vi "Main.vi"() -> ()   [LabVIEW 2020]
uses:
  System.Windows.Forms
  Global_Variable/Global.vi
  Global_Variable/A131258.vi
  Database/Global1.vi
  <userlib>/_MGI/Menu Building/MenuTypes/MenuStrip/MGI_MenuStrip.lvclass
  <userlib>/_MGI/Menu Building/MenuItemStatusChange/MGI_MenuItemStatusChange.lvclass
  Libraries/S7/S7.lvlib
panel:
  out "右加载扭矩":dbl format="%#.3f Nm"
  out "左空载扭矩":dbl format="%#.3f Nm"
  out "上序状态":string
  in  "表格控件":string[][](table)
  in  "Andon":enum32{"未选择", "缺料报警", "质量报警", "故障报警"}(radio)
  out "PLC":bool
  in  "菜单":refnum<k24>(container)
  out "试验计时":u16
  out "工位传感器码":string
  out "生产数量":i32
  out "合格数量":i32
  out "userStatus":string caption="用户状态"
  out "userName":string caption="用户名"
  out "connectionMode":string caption="联机类型"
  out "产品型号":string
  in  "更换产品":refnum<vi>
  out "提示信息":string
  out "错误":bool
  out "时间字符串":string
  out "日期字符串":string
  out "自动":bool
  # "芯轴分总成磨合台"
  # "试验项目"
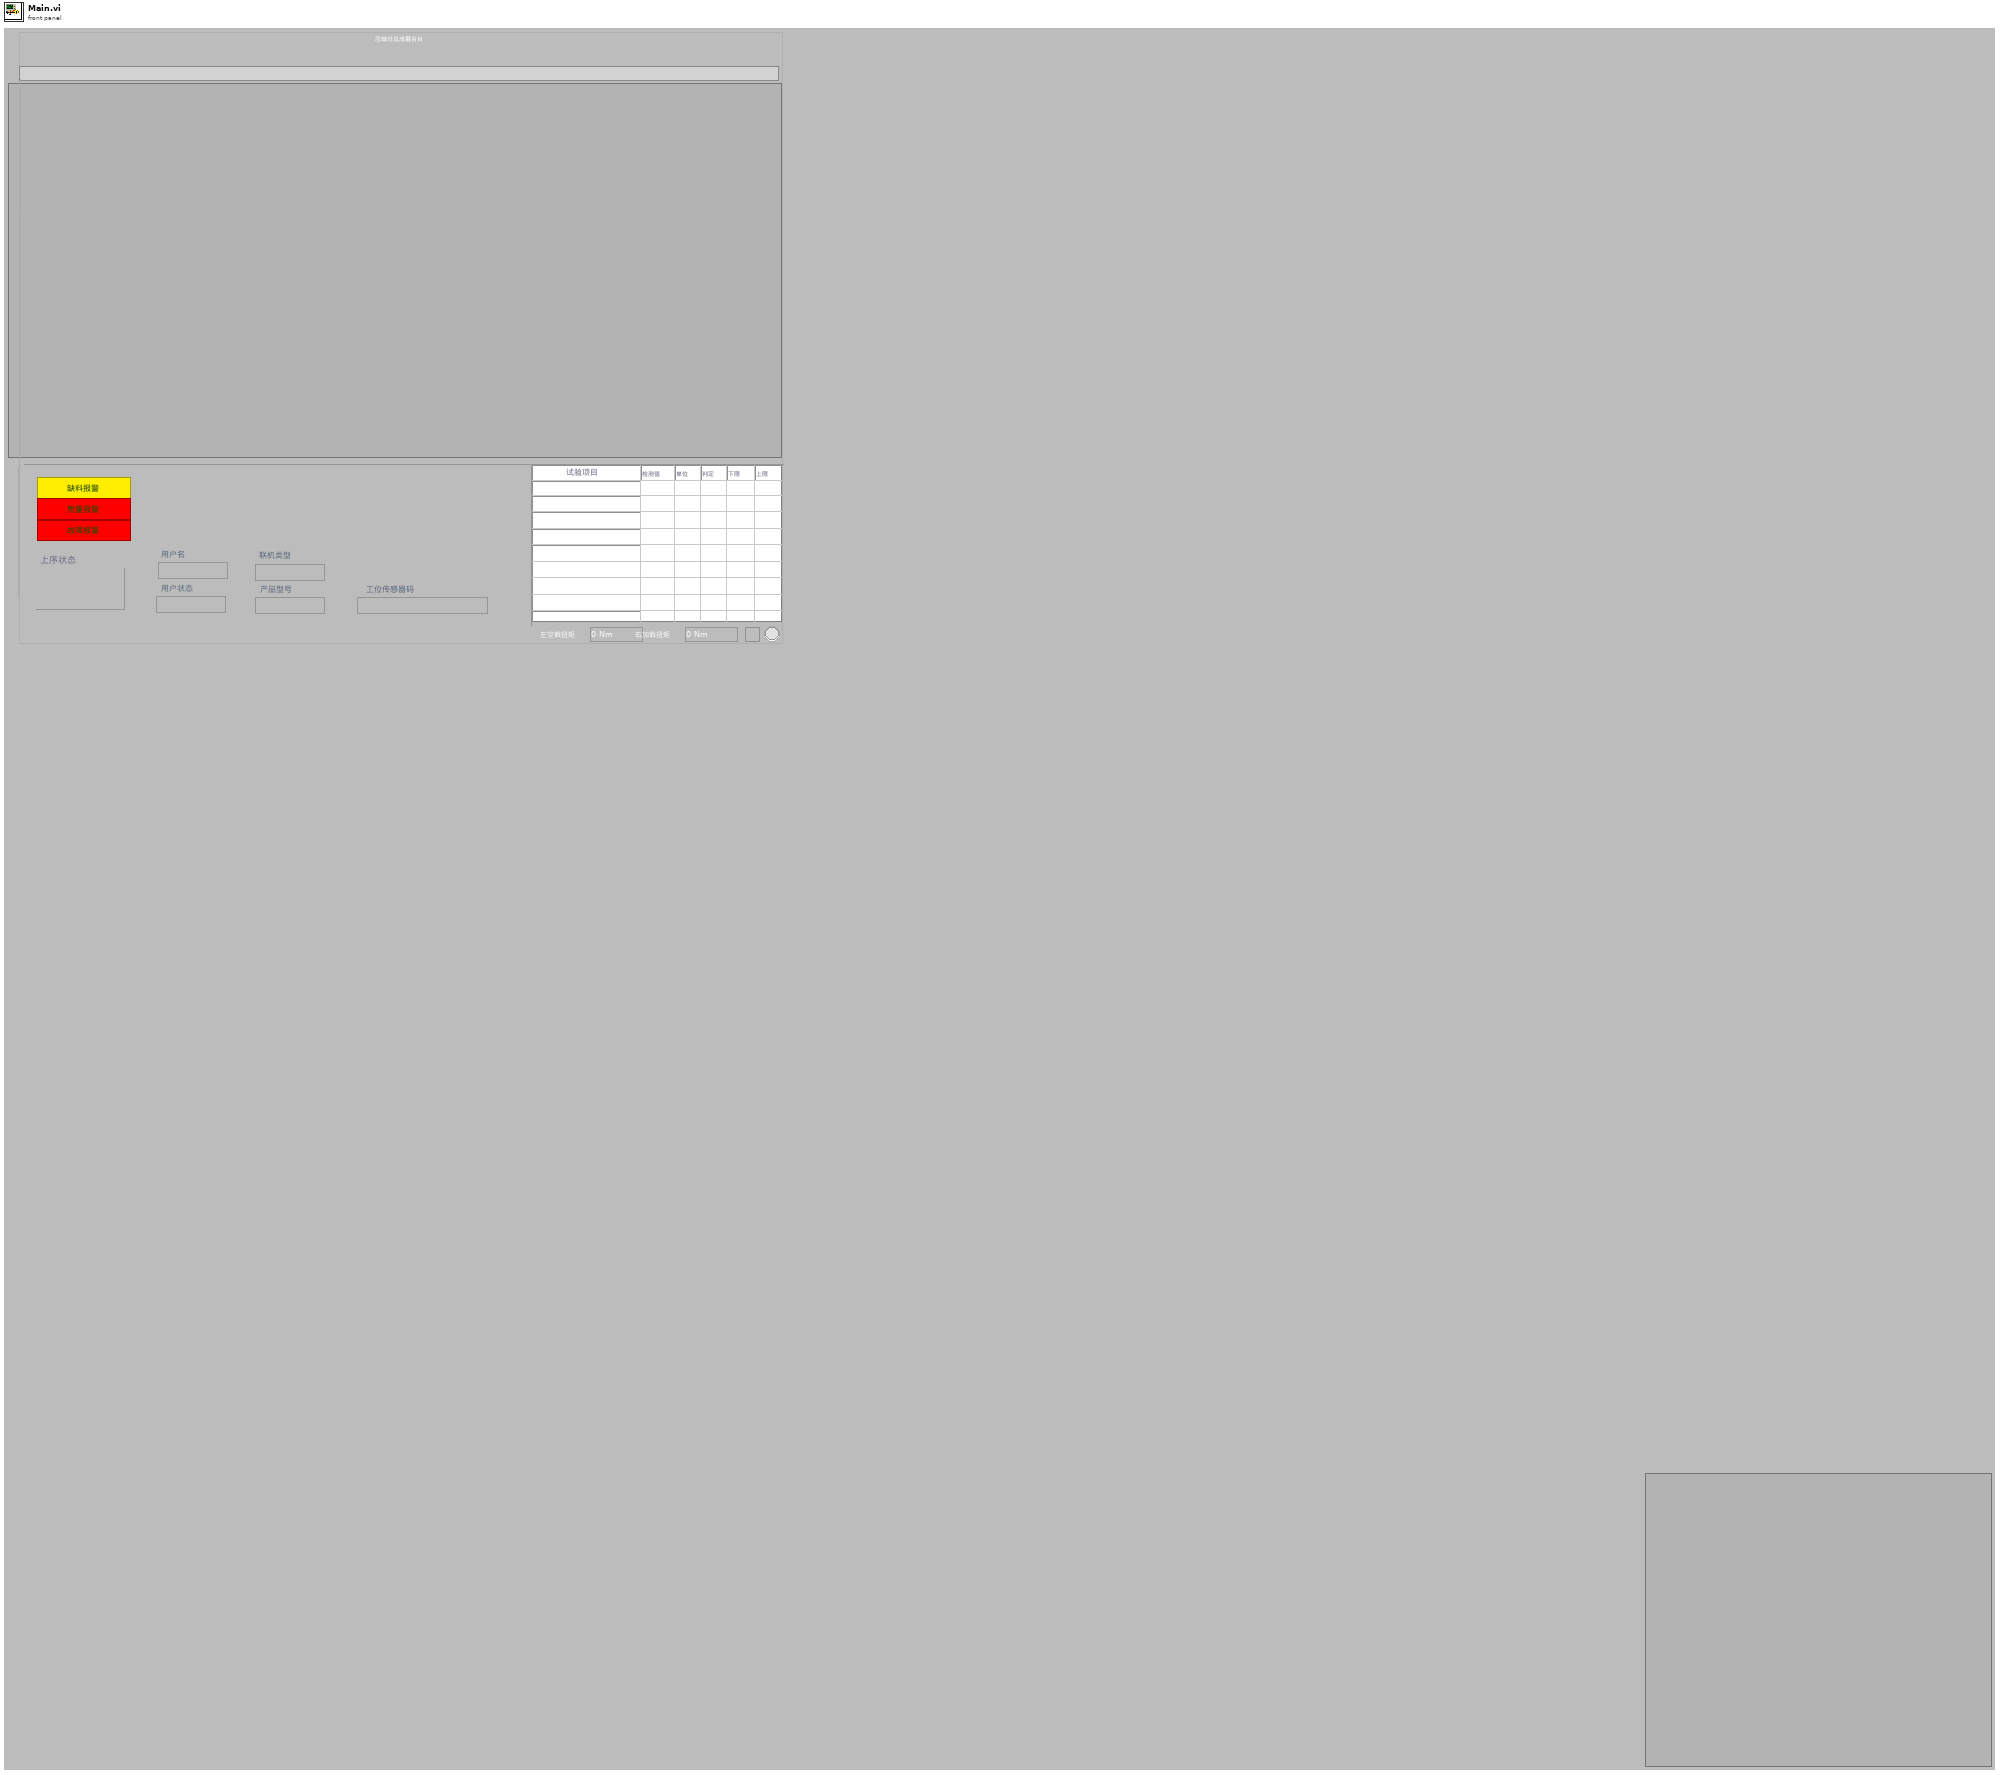
[diagram p1: front panel]
types:
  T1 = typedef "S7.lvlib/Broadcast Events--cluster.ctl" = cluster{"Module Did Init":refnum<user-event>, "Status Updated":refnum<user-event>, "Error Reported":refnum<user-event>, "Module Did Stop":refnum<user-event>, "Update Module Execution Status":refnum<user-event>}
  T2 = enum32{"Invalid", "Standard", "Closed", "Hidden", "Minimized", "Maximized"}
  T3 = cluster{"设备名称":string, "操作人员":string, "设备状态":enum16{"设备离线", "设备正常", "设备缺料", "设备故障", "质量报警"}, "附加信息":string}
  T4 = enum32{"invalid app kind", "Development System", "Run Time System", "Student Edition", "Embedded LabVIEW", "Evaluation", "Custom"}
  T5 = cluster{"左平均扭矩":cluster{"正转":dbl, "反转":dbl}, "左矩波动":cluster{"正转":dbl, "反转":dbl}, "左空载":cluster{"正转":dbl, "反转":dbl}, "右平均扭矩":cluster{"正转":dbl, "反转":dbl}, "右扭矩波动":cluster{"正转":dbl, "反转":dbl}, "右空载":cluster{"正转":dbl, "反转":dbl}, "扭矩对称":cluster{"左":dbl, "右":dbl}, "左零点漂移":cluster{"正":dbl, "反":dbl}, "右零点漂移":cluster{"正":dbl, "反":dbl}}
  T6 = cluster{"用户编号":string, "用户名":string, "用户密码(密文)":string, "用户权限":string}
  T7 = cluster{"Core":cluster{"Current VI Reference":refnum<vi>, "Close Panel on Exit?":bool}, "Your Boolean data":bool, "Your string data":string}
  T8 = cluster{"Current VI Reference":refnum<vi>, "Close Panel on Exit?":bool}
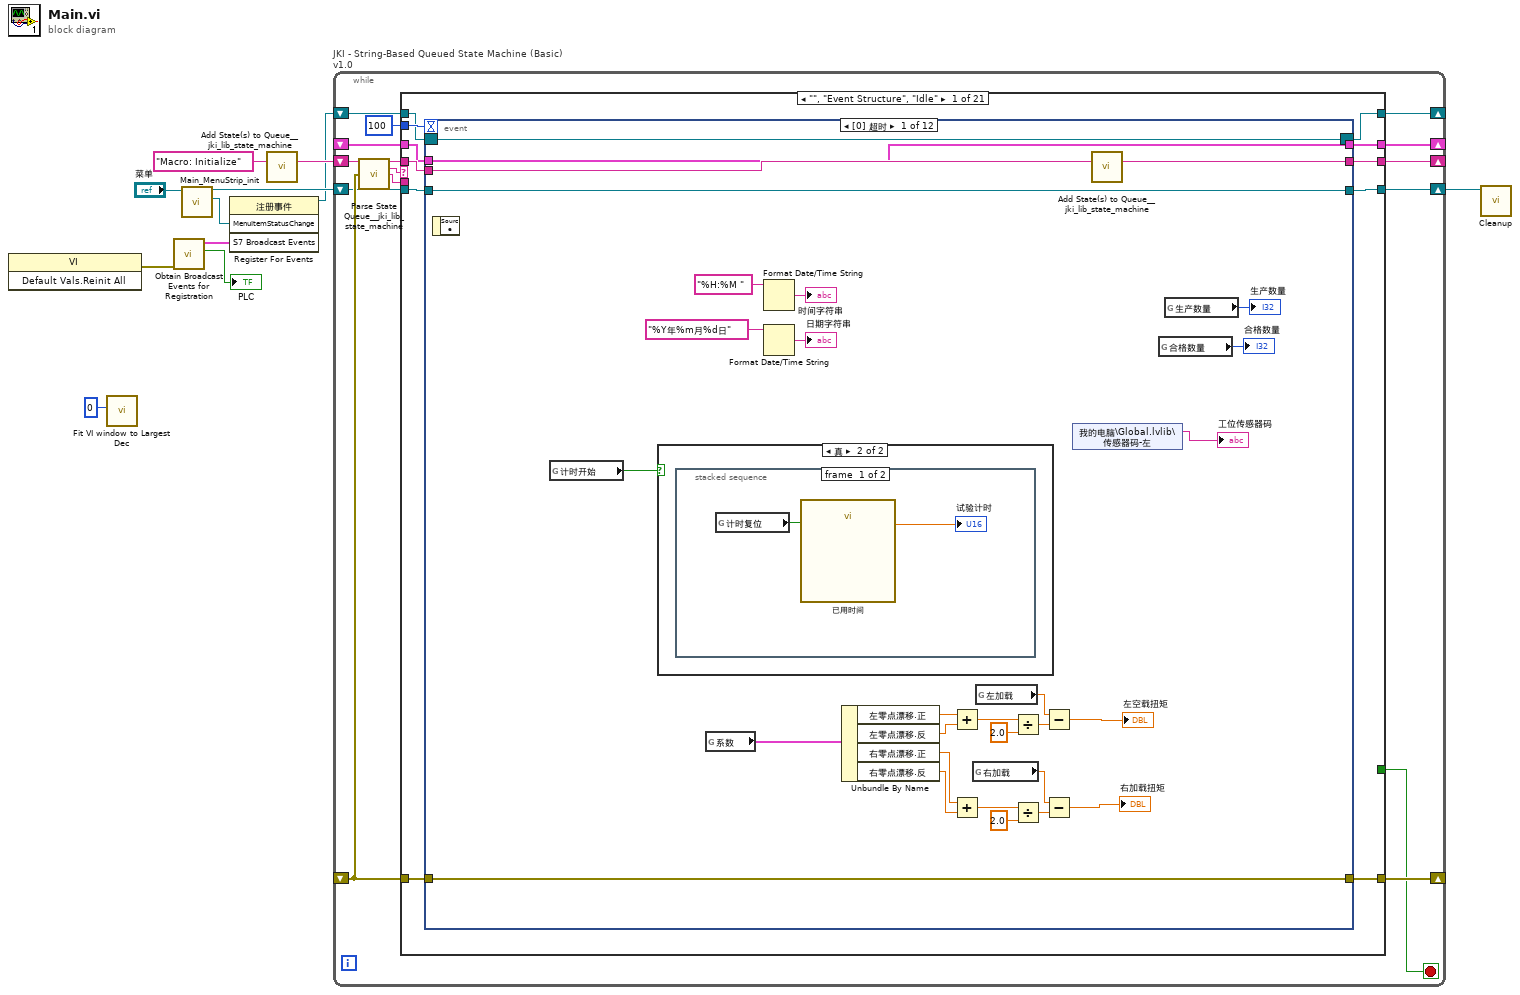
[diagram p0: block diagram]
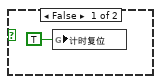
[diagram p2: hidden frame]
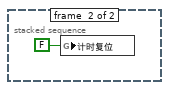
[diagram p3: hidden frame]
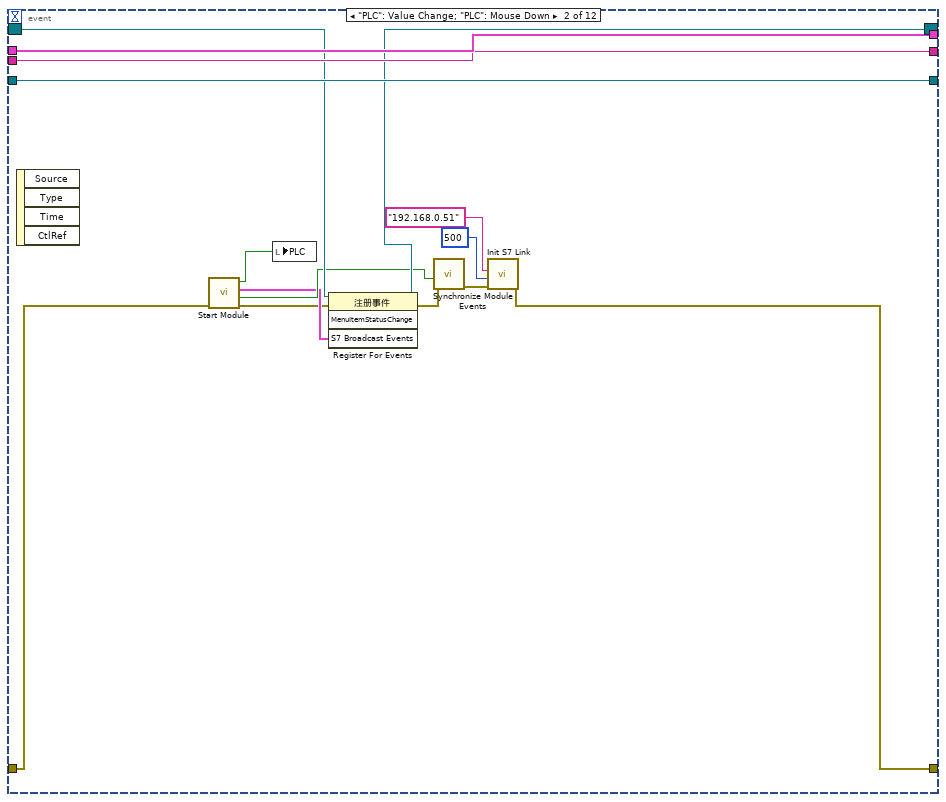
[diagram p4: hidden frame]
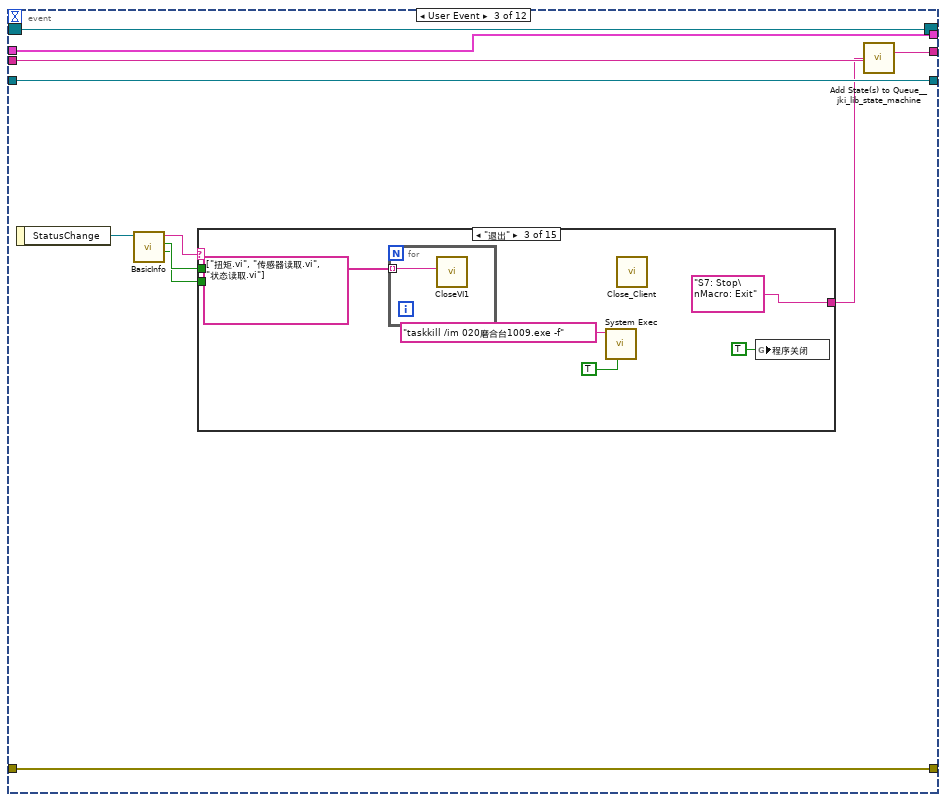
[diagram p5: hidden frame]
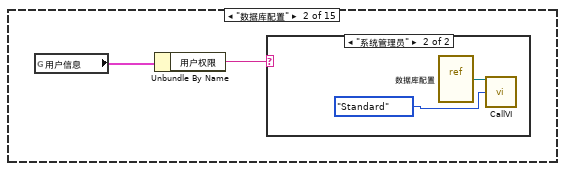
[diagram p7: hidden frame]
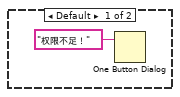
[diagram p8: hidden frame]
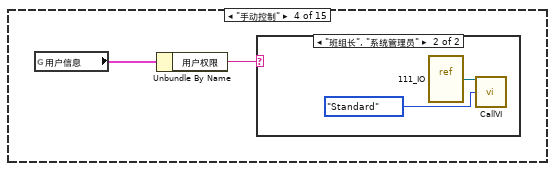
[diagram p9: hidden frame]
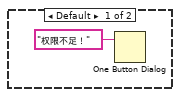
[diagram p10: hidden frame]
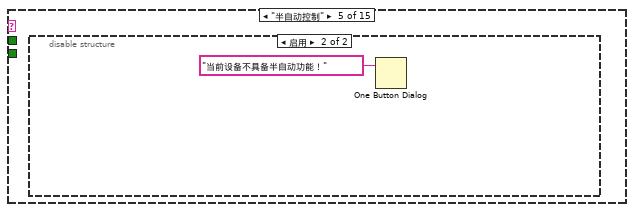
[diagram p11: hidden frame]
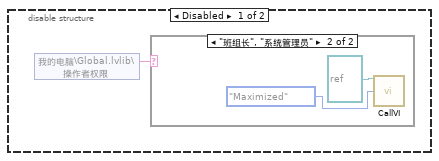
[diagram p12: hidden frame]
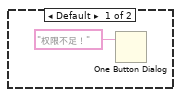
[diagram p13: hidden frame]
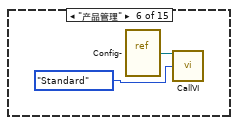
[diagram p14: hidden frame]
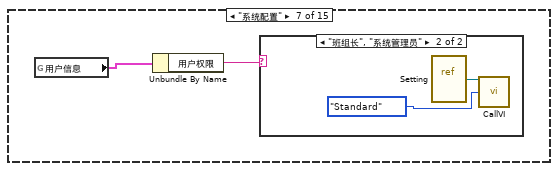
[diagram p15: hidden frame]
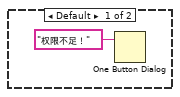
[diagram p16: hidden frame]
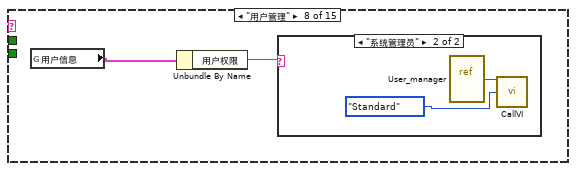
[diagram p17: hidden frame]
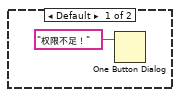
[diagram p18: hidden frame]
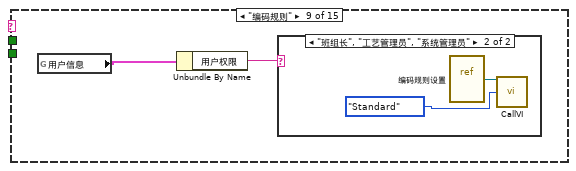
[diagram p19: hidden frame]
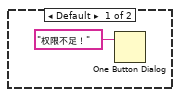
[diagram p20: hidden frame]
diagram:
  n1 = invoke class="VI" method="Default Vals.Reinit All"() -> (error out=w4:errorcluster)  [unwired: 3 in, 2 out]
  n2 = call "Fit VI window to Largest Dec.vi"("border spacing (2 px)"=0) -> ()  [unwired: 5 in, 2 out]
  n3 = call "Obtain Broadcast Events for Registration.vi"("error in (no error)"=w4) -> ("Already running?"=→"PLC":bool, "S7 Broadcast Events"=w6:T1)  [unwired: 8 in, 1 out]
  n4 = call "Main_MenuStrip_init.vi"("MenuStrip"="菜单") -> ("MenuItemStatusChange"=w3:refnum<user-event>, "Menu out"=w8:refnum<class "MGI_MenuStrip.lvclass">)  [unwired: 9 in]
  n5 = register-events(w3, w6) -> (reference out=w2:refnum<event-registration>)  [unwired: 2 in, 1 out]
  n6 = call <vilib>:"Add State(s) to Queue__jki_lib_state_machine.vi"("State(s) in (\"\")"="Macro: Initialize") -> ("States Out"=w11:string)  [unwired: 14 in]
  n7 = while "JKI - String-Based Queued State Machine (Basic) v1.0" {
    shift-right: [w20] -> _
    shift-left: _ -> [w19]
    shift-right: [w22] -> _
    shift-left: _ -> [w17]
    shift-right: [w21] -> _
    shift-left: w11 -> [w23]
    shift-right: [w15] -> w7
    shift-left: w8 -> [w16]
    shift-right: [w13] -> _
    shift-left: w2 -> [w12]
    stop <- w14 stop-if-true
    n8 = call <vilib>:"Parse State Queue__jki_lib_state_machine.vi"("State Queue"=w23, "Error In (no error)"=w17) -> ("Remaining States"=w25:string, "Current State"=w26:string, "Arguments"=w24:string)  [unwired: 11 in]
    n9 = case shown="\"\", \"Event Structure\", \"Idle\"" w26 {
      selector: w26 -> [_ _ w249 _ _ _ _ _ _ _ _ _ _ _ _ _ _ _ _ _ _]
      tunnel: w25 -> [w37 w246 w253 w273 w281 w289 w295 w299 w305 w314 w325 w333 w339 w349 w373 w409 w417 w430 w458 w465 w478]
      tunnel: w24 -> [_ _ _ _ _ _ _ _ _ _ _ _ _ _ _ _ w412 w424 _ _ _]
      tunnel: w19 -> [w35 w243 w251 w264 w278 w287 w292 w300 w308 w311 _ w328 w336 w347 w371 w406 w415 w426 w455 w462 w475]
      tunnel: [w34 w244 w255 w270 errorcluster {"status"=FALSE, "code"=0, "source"=""} ("error out") w286 w293 w297 w303 w312 w322 w329 w337 w346 w369 w407 w413 w427 w456 w463 w476] -> w22
      tunnel: w17 -> [w33 w244 w254 w270 w277 w286 w293 w297 w304 w312 w322 w330 w337 w340 w369 w407 w414 w428 w456 w463 w476]
      tunnel: [w36 w245 w252 w272 w280 w288 w294 w299 w306 w313 w324 w332 w338 w348 w372 w408 w416 w429 w457 w464 w477] -> w21
      tunnel: [w32 w243 w251 w271 w278 w287 w292 w300 w308 w311 w323 w328 w336 w347 w371 w406 w415 w426 w455 w462 w475] -> w20
      tunnel: 100 ("Timeout") -> [w31 _ _ _ _ _ _ _ _ _ _ _ _ _ _ _ _ _ _ _ _]
      tunnel: w16 -> [w30 w242 w248 w261 w275 w285 w291 w298 w307 w310 w317 w327 w335 w345 w370 w405 w411 w423 w454 w460 w468]
      tunnel: [w29 w242 w248 w261 w275 w285 w291 w298 w307 w310 w317 w327 w335 w345 w370 w405 w411 w423 w454 w460 w468] -> w15
      tunnel: [_ _ _ _ _ TRUE _ _ _ _ _ _ _ _ _ _ _ _ _ _ _] -> w14
      tunnel: [w27 w241 w247 w260 w274 w283 w290 w301 w302 w309 w318 w326 w334 w344 w368 w402 w410 w422 w453 w459 w467] -> w13
      tunnel: w12 -> [w28 w241 w247 w260 w274 w283 w290 w301 w302 w309 w318 w326 w334 w344 w368 w402 w410 w422 w453 w459 w467]
      frame "", "Event Structure", "Idle" {
        n10 = event shown="[0] 超时" {
          selector: w28 -> [w56 w80 w86 w156 w163 w170 w177 w191 w200 w208 w217 _]
          dyn-events: [w56 w79 w86 w156 w163 w170 w177 w191 w200 w208 w217 _] -> w27
          timeout: w31 -> [_ _ _ _ _ _ _ _ _ _ _ _]
          tunnel: w37 -> [w66 w84 w95 w157 w164 w173 w180 w188 w204 w215 w219 w235]
          tunnel: [w65 w84 w93 w158 w165 w174 w181 w189 w205 w214 w220 w235] -> w36
          tunnel: w35 -> [w64 w85 w94 w160 w168 w175 w182 w190 w206 w212 w222 w236]
          tunnel: [w57 w81 w96 w161 w166 w171 w183 w186 w203 w213 w221 w233] -> w34
          tunnel: w33 -> [w57 w82 w96 w161 w166 w171 w184 w186 w203 w213 w221 w233]
          tunnel: [w64 w85 w94 w160 w168 w175 w182 w190 w206 w212 w222 w236] -> w32
          tunnel: w30 -> [w55 w83 w89 w159 w167 w172 w179 w187 _ _ _ w234]
          tunnel: [w55 w83 w89 w159 w167 w172 w179 w187 _ _ _ w234] -> w29
          event Timeout {
            n11 = event-data() -> ()  [unwired: 1 in, 1 out]
            n12 = global read "Global.vi" "计时开始"() -> (w54:bool)
            n13 = case shown="真" w54 {
              frame False {
                n14 = global write "Global.vi" "计时复位"(TRUE ("计时复位")) -> ()
              }
              frame True {
                n15 = stacked-sequence {
                  frame #0 {
                    n16 = global read "Global.vi" "计时复位"() -> (w68:bool)
                    n17 = call "已用时间"("Reset"=w68) -> ("Elapsed Time (s)"=→"试验计时":dbl)  [unwired: 11 in, 7 out]
                  }
                  frame #1 {
                    n18 = global write "Global.vi" "计时复位"(FALSE ("计时复位")) -> ()
                  }
                }
              }
            }
            n19 = global read "A131258.vi" "系数"() -> (w38:T5)
            n20 = Format Date/Time String(time format string (%c)="%H:%M ") -> (date/time string=→"时间字符串":string)  [unwired: 2 in]
            n21 = Format Date/Time String(time format string (%c)="%Y年%m月%d日") -> (date/time string=→"日期字符串":string)  [unwired: 2 in]
            n22 = Unbundle By Name(w38) -> ("左零点漂移.正"=w39:dbl, "左零点漂移.反"=w40:dbl, "右零点漂移.正"=w47:dbl, "右零点漂移.反"=w48:dbl)
            n23 = Add(x=w39, y=w40) -> (x+y=w41:dbl)
            n24 = Add(x=w47, y=w48) -> (x+y=w46:dbl)
            n25 = global read "全局2.vi" "右加载"() -> (w49:dbl)
            n26 = global read "全局1.vi" "左加载"() -> (w43:dbl)
            n27 = Divide(x=w41, y=2.0) -> (x/y=w42:dbl)
            n28 = Divide(x=w46, y=2.0) -> (x/y=w45:dbl)
            n29 = Subtract(x=w43, y=w42) -> (x-y=→"左空载扭矩":dbl)
            n30 = Subtract(x=w49, y=w45) -> (x-y=→"右加载扭矩":dbl)
            n31 = shared-variable "我的电脑\\Global.lvlib\\传感器码-左"() -> (→"工位传感器码":string)  [unwired: 1 in, 1 out]
            n32 = call <vilib>:"Add State(s) to Queue__jki_lib_state_machine.vi"("State(s) in (\"\")"=w66) -> ("States Out"=w65:string)  [unwired: 14 in]
            n33 = global read "Global.vi" "合格数量"() -> (→"合格数量":i32)
            n34 = global read "Global.vi" "生产数量"() -> (→"生产数量":i32)
          }
          event "PLC": Value Change; "PLC": Mouse Down {
            n35 = event-data() -> ()  [unwired: 1 in, 4 out]
            n36 = call "Start Module.vi"("error in (no error)"=w82) -> ("error out"=w75:errorcluster, "Wait for Event Sync?"=w78:bool, "S7 Broadcast Events"=w77:T1, "Module Was Already Running?"=w76:bool)  [unwired: 7 in]
            n37 = local write "PLC"(w76) -> ()
            n38 = register-events(reference=w80, error in=w75, w77) -> (reference out=w79:refnum<event-registration>, error out=w74:errorcluster)  [unwired: 1 in]
            n39 = call "Synchronize Module Events.vi"("error in (no error)"=w74, "Wait for Event Sync?"=w78) -> ("error out"=w71:errorcluster)  [unwired: 9 in]
            n40 = call "Init S7 Link.vi"("error in (no error)"=w71, "超时"=500, "IP"="192.168.0.51") -> ("error out"=w81:errorcluster)  [unwired: 8 in]
          }
          event User Event {
            n41 = event-data() -> ("StatusChange"=w87:refnum<class "MGI_MenuItemStatusChange.lvclass">)  [unwired: 1 in]
            n42 = call <userlib>:"BasicInfo.vi"("MGI_MenuItemStatusChange in"=w87) -> ("Enabled?"=w90:bool, "Checked?"=w91:bool, "Tag"=w92:string)  [unwired: 7 in, 1 out]
            n43 = case shown="\"退出\"" w92 {
              tunnel: w91 -> [_ _ _ _ _ _ _ _ _ _ _ _ _ _ _]
              tunnel: w90 -> [_ _ _ _ _ _ _ _ _ _ _ _ _ _ _]
              tunnel: [_ _ "S7: Stop\nMacro: Exit" _ _ _ _ _ _ _ _ _ _ _ _] -> w88
              frame "假", Default {
              }
              frame "数据库配置" {
                n44 = global read "Global1.vi" "用户信息"() -> (w97:T6)
                n45 = Unbundle By Name(w97) -> ("用户权限"=w98:string)
                n46 = case shown="\"系统管理员\"" w98 {
                  frame Default {
                    n47 = One Button Dialog(message="权限不足！" ("消息")) -> ()  [unwired: 1 in, 1 out]
                  }
                  frame "系统管理员" {
                    n48 = vi-ref "数据库配置.vi"() -> (w101:refnum<vi>)
                    n49 = call "CallVI.vi"("VI引用"=w101, "状态"=T2."Standard") -> ()  [unwired: 11 in, 3 out]
                  }
                }
              }
              frame "退出" {
                n50 = for {
                  tunnel: string[] ["扭矩.vi", "传感器读取.vi", "状态读取.vi"] -> [w107] mode=indexing
                  n51 = call "CloseVI1.vi"("名称或相对路径"=w107) -> ()  [unwired: 10 in, 1 out]
                }
                n52 = call <vilib>:"System Exec.vi"("run minimized? (F)"=TRUE, "command line"="taskkill /im 020磨合台1009.exe -f") -> ()  [unwired: 6 in, 4 out]
                n53 = call "Close_Client.vi"() -> ()  [unwired: 12 in]
                n54 = global write "Global.vi" "程序关闭"(TRUE ("程序关闭")) -> ()
              }
              frame "手动控制" {
                n55 = global read "Global1.vi" "用户信息"() -> (w108:T6)
                n56 = Unbundle By Name(w108) -> ("用户权限"=w109:string)
                n57 = case shown="\"班组长\", \"系统管理员\"" w109 {
                  frame Default {
                    n58 = One Button Dialog(message="权限不足！" ("消息")) -> ()  [unwired: 1 in, 1 out]
                  }
                  frame "班组长", "系统管理员" {
                    n59 = vi-ref "111_IO.vi"() -> (w112:refnum<vi>)
                    n60 = call "CallVI.vi"("VI引用"=w112, "状态"=T2."Standard") -> ()  [unwired: 11 in, 3 out]
                  }
                }
              }
              frame "半自动控制" {
                n61 = disable-structure shown="启用" {
                  frame Disabled {
                    n62 = shared-variable "我的电脑\\Global.lvlib\\操作者权限"() -> (w113:string)  [unwired: 1 in, 1 out]
                    n63 = case shown="\"班组长\", \"系统管理员\"" w113 {
                      frame Default {
                        n64 = One Button Dialog(message="权限不足！" ("消息")) -> ()  [unwired: 1 in, 1 out]
                      }
                      frame "班组长", "系统管理员" {
                        n65 = call "CallVI.vi"("VI引用"=refnum<vi> refnum, "状态"=T2."Maximized") -> ()  [unwired: 11 in, 3 out]
                      }
                    }
                  }
                  frame Enabled {
                    n66 = One Button Dialog(message="当前设备不具备半自动功能！" ("消息")) -> ()  [unwired: 1 in, 1 out]
                  }
                }
              }
              frame "产品管理" {
                n67 = vi-ref "Config-.vi"() -> (w119:refnum<vi>)
                n68 = call "CallVI.vi"("VI引用"=w119, "状态"=T2."Standard") -> ()  [unwired: 11 in, 3 out]
              }
              frame "系统配置" {
                n69 = global read "Global1.vi" "用户信息"() -> (w120:T6)
                n70 = Unbundle By Name(w120) -> ("用户权限"=w121:string)
                n71 = case shown="\"班组长\", \"系统管理员\"" w121 {
                  frame Default {
                    n72 = One Button Dialog(message="权限不足！" ("消息")) -> ()  [unwired: 1 in, 1 out]
                  }
                  frame "班组长", "系统管理员" {
                    n73 = vi-ref "Setting.vi"() -> (w124:refnum<vi>)
                    n74 = call "CallVI.vi"("VI引用"=w124, "状态"=T2."Standard") -> ()  [unwired: 11 in, 3 out]
                  }
                }
              }
              frame "用户管理" {
                n75 = global read "Global1.vi" "用户信息"() -> (w125:T6)
                n76 = Unbundle By Name(w125) -> ("用户权限"=w126:string)
                n77 = case shown="\"系统管理员\"" w126 {
                  frame Default {
                    n78 = One Button Dialog(message="权限不足！" ("消息")) -> ()  [unwired: 1 in, 1 out]
                  }
                  frame "系统管理员" {
                    n79 = vi-ref "User_manager.vi"() -> (w129:refnum<vi>)
                    n80 = call "CallVI.vi"("VI引用"=w129, "状态"=T2."Standard") -> ()  [unwired: 11 in, 3 out]
                  }
                }
              }
              frame "编码规则" {
                n81 = global read "Global1.vi" "用户信息"() -> (w130:T6)
                n82 = Unbundle By Name(w130) -> ("用户权限"=w131:string)
                n83 = case shown="\"班组长\", \"工艺管理员\", \"系统管理员\"" w131 {
                  frame Default {
                    n84 = One Button Dialog(message="权限不足！" ("消息")) -> ()  [unwired: 1 in, 1 out]
                  }
                  frame "班组长", "工艺管理员", "系统管理员" {
                    n85 = vi-ref "编码规则设置.vi"() -> (w134:refnum<vi>)
                    n86 = call "CallVI.vi"("VI引用"=w134, "状态"=T2."Standard") -> ()  [unwired: 11 in, 3 out]
                  }
                }
              }
              frame "易损件管理" {
                n87 = vi-ref "易损件管理.vi"() -> (w136:refnum<vi>)
                n88 = call "CallVI.vi"("VI引用"=w136, "状态"=T2."Standard") -> ()  [unwired: 11 in, 3 out]
              }
              frame "物料批次管理" {
                n89 = vi-ref "批次管理.vi"() -> (w138:refnum<vi>)
                n90 = call "CallVI.vi"("VI引用"=w138, "状态"=T2."Standard") -> ()  [unwired: 11 in, 3 out]
              }
              frame "报表" {
                n91 = call "文件对话框"("start path"=path "D:/report", "prompt"="打开报表", "pattern (all files)"="*.doc;*.docx", "pattern label"="Word 文档") -> ("selected path"=w139:path, "error out"=w140:errorcluster)  [unwired: 8 in, 2 out]
                n92 = case shown="无错误" w140 {
                  selector: w140 -> [w146 w148]
                  tunnel: w139 -> [w147 _]
                  frame No Error {
                    w145 = 1 items=["Normal", "Maximize", "Minimize"] ("cpubbs_WindowState")
                    n93 = call "Open_Word.vi"("File Path"=w147, "cpubbs_WindowState"=w145, "错误输入（无错误）"=w146) -> ()  [unwired: 12 in, 1 out]
                  }
                  frame Error {
                    n94 = call <vilib>:"Clear Errors.vi"("error in (no error)"=w148) -> ()  [unwired: 5 in, 2 out]
                  }
                }
              }
              frame "报警信息" {
                n95 = vi-ref "报警信息.vi"() -> (w150:refnum<vi>)
                n96 = call "CallVI.vi"("VI引用"=w150, "状态"=T2."Standard") -> ()  [unwired: 11 in, 3 out]
              }
              frame "关于" {
                n97 = vi-ref "About.vi"() -> (w152:refnum<vi>)
                n98 = call "CallVI.vi"("VI引用"=w152, "状态"=T2."Standard") -> ()  [unwired: 11 in, 3 out]
              }
              frame "操作演示" {
                n99 = call <vilib>:"Application Directory.vi"() -> ("Application Directory"=w155:path)
                n100 = Build Path(base path=w155, name or relative path="操作演示" ("名称或相对路径")) -> (appended path=w154:path)
                n101 = call "自动播放ppt.vi"("路径"=w154) -> ()  [unwired: 10 in, 1 out]
              }
            }
            n102 = call <vilib>:"Add State(s) to Queue__jki_lib_state_machine.vi"("State(s) in (\"\")"=w95, "State(s) at Back (\"\")"=w88) -> ("States Out"=w93:string)  [unwired: 13 in]
          }
          event User Event {
            n103 = event-data() -> ("Init?"=w162:bool)  [unwired: 1 in, 1 out]
            n104 = local write "PLC"(w162) -> ()
            n105 = call <vilib>:"Add State(s) to Queue__jki_lib_state_machine.vi"("State(s) in (\"\")"=w157) -> ("States Out"=w158:string)  [unwired: 14 in]
          }
          event User Event {
            n106 = event-data() -> ("Running?"=w169:bool)  [unwired: 1 in]
            n107 = local write "PLC"(w169) -> ()
            n108 = call <vilib>:"Add State(s) to Queue__jki_lib_state_machine.vi"("State(s) in (\"\")"=w164) -> ("States Out"=w165:string)  [unwired: 14 in]
          }
          event User Event {
            n109 = event-data() -> ()  [unwired: 1 in, 7 out]
            n110 = local write "PLC"(FALSE ("PLC")) -> ()
            n111 = call <vilib>:"Add State(s) to Queue__jki_lib_state_machine.vi"("State(s) in (\"\")"=w173) -> ("States Out"=w174:string)  [unwired: 14 in]
          }
          event User Event {
            n112 = event-data() -> ("Error"=w185:errorcluster)  [unwired: 1 in]
            n113 = Merge Errors(w185, w184) -> (w183:errorcluster)
            n114 = call <vilib>:"Add State(s) to Queue__jki_lib_state_machine.vi"("State(s) in Front (\"\")"="S7: Initialize\nIdle", "State(s) in (\"\")"=w180) -> ("States Out"=w181:string)  [unwired: 13 in]
          }
          event "自动": Mouse Down {
            n115 = event-data() -> ()  [unwired: 1 in, 1 out]
            n116 = disable-structure shown="禁用" {
              frame Disabled {
                n117 = local read "自动"() -> (w192:bool)
                n118 = case shown="假" w192 {
                  frame False {
                    n119 = call "设备状态.vi"() -> ("Status_Read"=w193:i16)  [unwired: 11 in]
                    n120 = case shown="5" w193 {
                      frame 0, Default {
                        n121 = One Button Dialog(message="请复位！" ("消息")) -> ()  [unwired: 1 in, 1 out]
                      }
                      frame 5 {
                      }
                    }
                  }
                  frame True {
                    n122 = Two Button Dialog(message="确定要退出自动？" ("消息")) -> (T button?=w195:bool)  [unwired: 2 in]
                    n123 = case shown="真" w195 {
                      frame False {
                      }
                      frame True {
                        n124 = vi-ref "Auto - 副本.vi"() -> (w199:refnum<vi>)
                        n125 = invoke class="VI" method="Ctrl Val.Set"(reference=w199, "Control Name"="STEP" ("控件名"), "Value"="退出自动" ("控件名")) -> ()  [unwired: 2 in, 5 out]
                      }
                    }
                  }
                }
              }
              frame Enabled {
              }
            }
            n126 = call <vilib>:"Add State(s) to Queue__jki_lib_state_machine.vi"("State(s) in (\"\")"=w188) -> ("States Out"=w189:string)  [unwired: 14 in]
          }
          event "错误": Mouse Down {
            n127 = event-data() -> ()  [unwired: 1 in, 8 out]
            n128 = vi-ref "报警信息.vi"() -> (w202:refnum<vi>)
            n129 = call "CallVI.vi"("VI引用"=w202, "状态"=T2."Standard") -> ()  [unwired: 11 in, 3 out]
            n130 = call <vilib>:"Add State(s) to Queue__jki_lib_state_machine.vi"("State(s) in (\"\")"=w204) -> ("States Out"=w205:string)  [unwired: 14 in]
          }
          event Panel Close? {
            n131 = event-data() -> ()  [unwired: 1 in, 1 out]
            n132 = global write "Global.vi" "计时开始"(FALSE ("计时复位")) -> ()
            n133 = global write "Global.vi" "程序关闭"(TRUE ("程序关闭")) -> ()
            n134 = call <vilib>:"Add State(s) to Queue__jki_lib_state_machine.vi"("State(s) in Front (\"\")"="S7: Stop\nMacro: Exit", "State(s) in (\"\")"=w215) -> ("States Out"=w214:string)  [unwired: 13 in]
            n135 = event-data("Discard?"=TRUE) -> ()  [unwired: 1 in, 1 out]
          }
          event "更换产品": Value Change {
            n136 = event-data() -> ("NewVal"=w218:refnum<vi>)  [unwired: 1 in, 5 out]
            n137 = stacked-sequence {
              tunnel: w218 -> [w225]
              tunnel: ["Idle"] -> w216
              frame #0 {
                n138 = disable-structure shown="禁用" {
                  disable-tunnel: w225 -> [w227 _]
                  frame Disabled {
                    n139 = control-ref of="子面板"() -> (w226:refnum<vi>)
                    n140 = call "Call_SubPanal.vi"("VI引用句柄"=w227, "SubPnl引用句柄"=w226) -> ()  [unwired: 9 in, 1 out]
                  }
                  frame Enabled {
                  }
                }
                n141 = shared-variable "我的电脑\\Global.lvlib\\产品型号"() -> (w224:string)  [unwired: 1 in, 1 out]
                n142 = local write "产品型号"(w224) -> ()
              }
            }
            n143 = call <vilib>:"Add State(s) to Queue__jki_lib_state_machine.vi"("State(s) in Front (\"\")"=w216, "State(s) in (\"\")"=w219) -> ("States Out"=w220:string)  [unwired: 13 in]
          }
          event "Andon": Value Change {
            n144 = event-data() -> ("NewVal"=w232:enum32{"未选择", "缺料报警", "质量报警", "故障报警"})  [unwired: 1 in]
            n145 = case shown="\"故障报警\"" w232 {
              tunnel: [enum16{"设备离线", "设备正常", "设备缺料", "设备故障", "质量报警"}."设备正常" ("设备状态") enum16{"设备离线", "设备正常", "设备缺料", "设备故障", "质量报警"}."设备缺料" ("设备状态") enum16{"设备离线", "设备正常", "设备缺料", "设备故障", "质量报警"}."质量报警" ("设备状态") enum16{"设备离线", "设备正常", "设备缺料", "设备故障", "质量报警"}."设备故障" ("设备状态")] -> w230
              frame "未选择", Default {
              }
              frame "缺料报警" {
              }
              frame "质量报警" {
              }
              frame "故障报警" {
              }
            }
            n146 = local read "userName"() -> (w229:string)
            n147 = Bundle By Name(cluster=T3 {"设备名称"="芯轴分总成磨合台", "操作人员"="", "设备状态"=enum."设备离线", "附加信息"=""} ("设备信息"), "操作人员"=w229, "设备状态"=w230) -> (w228:T3)
            n148 = call "Change_Client.vi"("设备信息"=w228) -> ()  [unwired: 10 in, 1 out]
          }
        }
      }
      frame "---------- Core ----------" {
        n149 = call <vilib>:"Add State(s) to Queue__jki_lib_state_machine.vi"("State(s) in (\"\")"=w246) -> ("States Out"=w245:string)  [unwired: 14 in]
      }
      frame Default {
        w258 = 42 items=["No error", "Argument error", "Memory is full", "Out of zone", "End of file", "File already open", "Generic file I/O error", "File not found", "File permission error", "Disk is full", "Duplicate path", "Too many files open", "System feature not enabled", "Resource file not found", "Cannot add resource", "Resource not found", "Image not found", "Image memory error", "Pen does not exist", "Config type invalid", "Config token not found", "Config parse error", "Config memory error", "Bad external code format", "Bad external code offset", "External code not present", "Null window", "Destroy window error", "Null menu", "Print aborted", "Bad print record", "Print driver error", "Windows error during printing", "Memory error during printing", "Print dialog error", "Generic print error", "Invalid device refnum", "Device not found", "Device parameter error", "Device unit error", "Cannot open device", "Device call aborted", "Generic error", "Cancelled by user", "Object ID too low", "Object ID too high", "Object not in heap", "Unknown heap", "Unknown object (invalid DefProc)", "Unknown object (DefProc not in table)", "Message out of range", "Invalid (null) method", "Unknown message", "Manager call not supported", "Bad address", "Network operation in progress", "Network operation timed out", "Connection is busy", "Network attribute not supported", "Network error", "Address in use", "System out of memory", "Connection aborted", "Connection refused", "Not connected", "Already connected", "Connection closed", "Initialization error (interapplication manager)", "Bad occurrence", "Wait on unbound occurrence handler", "Occurrence queue overflow", "Datalog type conflict", "Unused", "Unrecognized type (interapplication manager)", "Memory corrupt", "Failed to make temporary DLL", "Old CIN version", "Drag socket not found", "Failed to load drop-object", "Failed to register OLE object", "Failed to release OLE object", "Format specifier type mismatch", "Unknown format specifier", "Too few format specifiers", "Too many format specifiers", "Scan failed", "Newer CIN version", "Error converting to variant", "Runtime menu error", "Password tampered", "Variant attribute not found", "Incompatible variant data type", "Event data is not available", "Event Store is not present", "Occurrence is not found", "Event Queue is not created", "Event info is not available", "Refnum passed is NULL", "Error retrieving Class GUID", "Error retrieving CoClass GUID", "Error retrieving TypeLib GUID.", "Bad built application magic bytes.", "Specific driver is different from the specific driver associated with the Logical Name.", "There is no session opened to the class driver.", "Max Error", "MAX - Error with config objects", "MAX - Error loading configuration", "MAX - Group not supported"]
        # "Current State"
        n150 = Format Into String(format string="Software Exception: Unhandled State \"%s\"." ("message"), error in=w254, w249) -> (resulting string=w257:string, error out=w256:errorcluster)  [unwired: 1 in]
        n151 = call <vilib>:"Error Cluster From Error Code.vi"("show call chain? (False)"=TRUE, "error in (no error)"=w256, "error message (\"\")"=w257, "error code (0)"=w258) -> ("error out"=w255:errorcluster)  [unwired: 5 in]
        n152 = call <vilib>:"Add State(s) to Queue__jki_lib_state_machine.vi"("State(s) in (\"\")"=w253) -> ("States Out"=w252:string)  [unwired: 14 in]
      }
      frame "Initialize Core Data" {
        # "originally closed?"
        # "exe?"
        n153 = property class="VI"() -> ("Front Panel.Open"=w269:bool)  [unwired: 2 in, 2 out]
        n154 = property class="App"() -> ("App.Kind"=w268:T4)  [unwired: 2 in, 2 out]
        n155 = control-ref of="Current VI Reference"() -> (w262:refnum<vi>)
        n156 = Not(x=w269) -> (.not. x?=w266:bool)
        n157 = Equal?(x=w268, y=T4."Run Time System" ("Application:Kind")) -> (x = y?=w265:bool)
        n158 = Or(x=w266, y=w265) -> (x .or. y?=w263:bool)
        n159 = Bundle By Name(cluster=w264, "Core.Current VI Reference"=w262, "Core.Close Panel on Exit?"=w263) -> (w271:T7)
        n160 = call <vilib>:"Add State(s) to Queue__jki_lib_state_machine.vi"("State(s) in (\"\")"=w273) -> ("States Out"=w272:string)  [unwired: 14 in]
      }
      frame "Error Handler" {
        n161 = call <vilib>:"General Error Handler.vi"("error in (no error)"=w277) -> ()  [unwired: 10 in, 5 out]
        n162 = call <vilib>:"Add State(s) to Queue__jki_lib_state_machine.vi"("State(s) in Front (\"\")"="/* Post Error States", "State(s) in (\"\")"=w281) -> ("States Out"=w280:string)  [unwired: 13 in]
      }
      frame "Exit" {
        n163 = call <vilib>:"Add State(s) to Queue__jki_lib_state_machine.vi"("State(s) in (\"\")"=w289) -> ("States Out"=w288:string)  [unwired: 14 in]
        n164 = Quit LabVIEW(quit? (T)=TRUE ("退出？(T)")) -> ()
      }
      frame "--------- Library --------" {
        n165 = call <vilib>:"Add State(s) to Queue__jki_lib_state_machine.vi"("State(s) in (\"\")"=w295) -> ("States Out"=w294:string)  [unwired: 14 in]
      }
      frame "S7: Initialize" {
        n166 = property on="PLC" class="Bool (严格)"("Val(Sgnl)"=FALSE ("值(信号)")) -> ()  [unwired: 2 in, 2 out]
      }
      frame "S7: Stop" {
        n167 = call "Stop Module.vi"("error in (no error)"=w304) -> ("error out"=w303:errorcluster)  [unwired: 10 in]
        n168 = call <vilib>:"Add State(s) to Queue__jki_lib_state_machine.vi"("State(s) in (\"\")"=w305) -> ("States Out"=w306:string)  [unwired: 14 in]
      }
      frame "---------- Data ----------" {
        n169 = call <vilib>:"Add State(s) to Queue__jki_lib_state_machine.vi"("State(s) in (\"\")"=w314) -> ("States Out"=w313:string)  [unwired: 14 in]
      }
      frame "Data: Initialize" {
        w319 = T8 {"Current VI Reference"=refnum, "Close Panel on Exit?"=FALSE}  # Core
        w321 = TRUE  # Your Boolean data
        w320 = ""  # Your string data
        n170 = global write "Global.vi" "程序关闭"(FALSE ("程序关闭")) -> ()
        n171 = global write "Global.vi" "计时开始"(FALSE ("计时结束")) -> ()
        n172 = Bundle("Core"=w319, "Your Boolean data"=w321, "Your string data"=w320) -> (w323:T7)  [unwired: 1 in]
        n173 = call <vilib>:"Add State(s) to Queue__jki_lib_state_machine.vi"("State(s) in (\"\")"=w325) -> ("States Out"=w324:string)  [unwired: 14 in]
      }
      frame "Data: Cleanup" {
        n174 = Unbundle By Name(w328) -> ("Core.Current VI Reference"=w331:refnum<vi>)
        n175 = Close Reference(reference=w331, error in (no error)=w330) -> (error out=w329:errorcluster)
        n176 = call <vilib>:"Add State(s) to Queue__jki_lib_state_machine.vi"("State(s) in (\"\")"=w333) -> ("States Out"=w332:string)  [unwired: 14 in]
      }
      frame "---------- UI ----------" {
        # "Do not put any code in this frame.\n(It is a separator no-op. You can make a copy of this frame to create a new UI frame)"
        n177 = call <vilib>:"Add State(s) to Queue__jki_lib_state_machine.vi"("State(s) in (\"\")"=w339) -> ("States Out"=w338:string)  [unwired: 14 in]
      }
      frame "UI: Initialize" {
        n178 = vi-ref "Auto.vi"() -> (w343:refnum<vi>)
        n179 = invoke class="VI" method="Ctrl Val.Set"(reference=w343, "Control Name"="STEP" ("控件名"), "Value"="初始化" ("控件名")) -> ()  [unwired: 2 in, 5 out]
        n180 = disable-structure shown="启用" {
          disable-tunnel: [w356 _] -> w346
          disable-tunnel: w340 -> [w354 _]
          frame Enabled {
            n181 = vi-ref "Auto.vi"() -> (w355:refnum<vi>)
            n182 = property class="VI"(reference=w355) -> (reference out=w353:refnum<vi>, "FP.State"=w352:T2)  [unwired: 1 in, 1 out]
            n183 = case shown="\"Standard\", 默认" w352 {
              tunnel: w354 -> [w362 w364]
              tunnel: w353 -> [w363 w365]
              tunnel: [w361 w365] -> w350
              tunnel: [w360 w364] -> w351
              frame "Standard", Default {
                n184 = invoke class="VI" method="FP.Close"(reference=w363, error in=w362) -> (reference out=w361:refnum<vi>, error out=w360:errorcluster)  [unwired: 1 in, 1 out]
              }
              frame "Invalid", "Closed" {
              }
            }
            n185 = invoke on="子面板" class="SubPnl" method="Insert VI"(error in=w351, "VI Ref"=w350) -> (error out=w359:errorcluster)  [unwired: 2 in, 3 out]
            n186 = invoke class="VI" method="Run VI"(reference=w350, error in=w359, "Wait until done"=FALSE ("结束前等待"), "Auto Dispose Ref"=TRUE ("自动销毁引用")) -> (error out=w356:errorcluster)  [unwired: 1 in, 4 out]
          }
          frame Disabled {
            n187 = vi-ref "Auto - 副本.vi"() -> (w367:refnum<vi>)
            n188 = call "CallVI.vi"("VI引用"=w367, "状态"=T2."Maximized") -> ()  [unwired: 11 in, 3 out]
          }
        }
        n189 = call <vilib>:"Add State(s) to Queue__jki_lib_state_machine.vi"("State(s) in (\"\")"=w349) -> ("States Out"=w348:string)  [unwired: 14 in]
      }
      frame "UI: Init" {
        n190 = stacked-sequence {
          tunnel: w369 -> [_ _ _ _]
          frame #0 {
            n191 = global write "Global.vi" "程序关闭"(FALSE ("程序关闭")) -> ()
            n192 = vi-ref "状态读取.vi"() -> (w378:refnum<vi>)
            n193 = vi-ref "扭矩.vi"() -> (w377:refnum<vi>)
            n194 = call "CallVI.vi"("VI引用"=w378, "状态"=T2."Hidden") -> ("错误输出"=w376:errorcluster)  [unwired: 11 in, 2 out]
            n195 = call "CallVI.vi"("VI引用"=w377, "状态"=T2."Hidden", "错误输入"=w376) -> ()  [unwired: 10 in, 3 out]
          }
          frame #1 {
            w386 = 0
            n196 = shared-variable "我的电脑\\Global.lvlib\\总成追溯码"("   " ("工位追溯码")) -> ()  [unwired: 1 in, 1 out]
            n197 = global write "Global.vi" "生产数量"(w386) -> ()
            n198 = global write "Global.vi" "合格数量"(w386) -> ()
            n199 = global read "Global1.vi" "用户信息"() -> (w381:T6)
            n200 = global read "Global1.vi" "联机模式"() -> (w380:enum16{"单机", "追溯"})
            n201 = Unbundle By Name(w381) -> ("用户名"=→"userName":string, "用户权限"=→"userStatus":string)
            n202 = case shown="\"追溯\"" w380 {
              tunnel: ["联网" ("connectionMode") "单机" ("connectionMode")] -> w387
              frame "追溯" {
              }
              frame "单机", Default {
              }
            }
            "connectionMode" <- w387
            "产品型号" <- "" ("产品型号")
          }
          frame #2 {
            n203 = control-ref of="表格控件"() -> (w391:refnum<vi>)
            n204 = control-ref of="提示信息"() -> (w393:refnum<vi>)
            n205 = control-ref of="自动"() -> (w394:refnum<vi>)
            n206 = control-ref of="错误"() -> (w395:refnum<vi>)
            n207 = control-ref of="更换产品"() -> (w392:refnum<vi>)
            n208 = global write "Global.vi" "提示信息"(w393) -> ()
            n209 = global write "Global.vi" "程序自动"(w394) -> ()
            n210 = global write "Global.vi" "报警图标"(w395) -> ()
            n211 = global write "Global.vi" "Result"(w391) -> ()
            n212 = global write "Global.vi" "更换产品"(w392) -> ()
            n213 = control-ref of="上序状态"() -> (w390:refnum<vi>)
            n214 = global write "Global.vi" "上序状态"(w390) -> ()
          }
          frame #3 {
            w396 = -2
            n215 = global read "Global.vi" "Result"() -> (w399:refnum<vi>)
            n216 = property class="Tbl"(reference=w399, "Row Headers[]"=string[] [], "Value"=string[][] []) -> ()  [unwired: 1 in, 2 out]
            n217 = Bundle(w396, w396) -> (w397:cluster{i32, i32})  [unwired: 1 in]
            n218 = call "Start_Client.vi"() -> ()  [unwired: 12 in]
            n219 = property class="Tbl"(reference=w399, "Active Cell"=w397, "Cell BG Color"=u32 16777216 ("活动单元格:单元格背景色")) -> ()  [unwired: 1 in, 2 out]
          }
        }
        n220 = call <vilib>:"Add State(s) to Queue__jki_lib_state_machine.vi"("State(s) in (\"\")"=w373) -> ("States Out"=w372:string)  [unwired: 14 in]
      }
      frame "UI: Config" {
        n221 = vi-ref "Config-.vi"() -> (w404:refnum<vi>)
        n222 = call "CallVI.vi"("VI引用"=w404, "状态"=T2."Standard") -> ()  [unwired: 11 in, 3 out]
        n223 = call <vilib>:"Add State(s) to Queue__jki_lib_state_machine.vi"("State(s) in (\"\")"=w409) -> ("States Out"=w408:string)  [unwired: 14 in]
      }
      frame "UI: Cursor Set" {
        # "Argument"
        n224 = case shown="\"Idle\", 默认" w412 {
          tunnel: w414 -> [w419 w421]
          tunnel: [w418 w420] -> w413
          frame "Idle", Default {
            n225 = call <vilib>:"Unset Busy.vi"("error in (no error)"=w419) -> ("error out"=w418:errorcluster)  [unwired: 10 in]
          }
          frame "Busy" {
            n226 = call <vilib>:"Set Busy.vi"("error in (no error)"=w421) -> ("error out"=w420:errorcluster)  [unwired: 9 in, 1 out]
          }
        }
        n227 = call <vilib>:"Add State(s) to Queue__jki_lib_state_machine.vi"("State(s) in (\"\")"=w417) -> ("States Out"=w416:string)  [unwired: 14 in]
      }
      frame "UI: Front Panel State" {
        # "Argument"
        n228 = Unbundle By Name(w426) -> ("Core.Current VI Reference"=w425:refnum<vi>)
        n229 = case shown="\"Close\"" w424 {
          tunnel: w428 -> [w434 w447]
          tunnel: [w436 w448] -> w427
          tunnel: w425 -> [w435 w445]
          frame "Open", Default {
            n230 = property class="VI"(reference=w435, error in=w434) -> (reference out=w432:refnum<vi>, error out=w433:errorcluster, "Front Panel.Open"=w431:bool)
            n231 = case shown="假" w431 {
              tunnel: [w439 w442] -> w436
              tunnel: w433 -> [w438 w442]
              tunnel: w432 -> [w437 _]
              frame False {
                n232 = invoke class="VI" method="FP.Open"(reference=w437, error in=w438, "Activate"=TRUE, "State"=T2."Standard") -> (error out=w439:errorcluster)  [unwired: 1 in, 4 out]
              }
              frame True {
              }
            }
          }
          frame "Close" {
            n233 = property class="VI"(reference=w445, error in=w447) -> (reference out=w444:refnum<vi>, error out=w446:errorcluster, "Front Panel.Open"=w443:bool)
            n234 = case shown="真" w443 {
              tunnel: [w449 w452] -> w448
              tunnel: w446 -> [w449 w451]
              tunnel: w444 -> [_ w450]
              frame False {
              }
              frame True {
                n235 = invoke class="VI" method="FP.Close"(reference=w450, error in=w451) -> (error out=w452:errorcluster)  [unwired: 1 in, 2 out]
              }
            }
          }
        }
        n236 = call <vilib>:"Add State(s) to Queue__jki_lib_state_machine.vi"("State(s) in (\"\")"=w430) -> ("States Out"=w429:string)  [unwired: 14 in]
      }
      frame "---------- Macro ----------" {
        n237 = call <vilib>:"Add State(s) to Queue__jki_lib_state_machine.vi"("State(s) in (\"\")"=w458) -> ("States Out"=w457:string)  [unwired: 14 in]
      }
      frame "Macro: Initialize" {
        n238 = call <vilib>:"Add State(s) to Queue__jki_lib_state_machine.vi"("State(s) in Front (\"\")"="Data: Initialize\nInitialize Core Data\nS7: Initialize\nIdle\nUI: Init\nUI: Front Panel State >> Open\nUI: Initialize\nUI: Config", "State(s) in (\"\")"=w465) -> ("States Out"=w464:string)  [unwired: 13 in]
      }
      frame "Macro: Exit" {
        n239 = Unbundle By Name(w475) -> ("Core.Close Panel on Exit?"=w474:bool)
        n240 = Select(t="UI: Front Panel State >> Close", s=w474, f="") -> (s? t:f=w471:string)
        n241 = call <vilib>:"Add State(s) to Queue__jki_lib_state_machine.vi"("State(s) in (\"\")"=w471, "State(s) at Back (\"\")"="Data: Cleanup\nExit") -> ("States Out"=w469:string)  [unwired: 13 in]
        n242 = Quit LabVIEW(quit? (T)=TRUE ("退出？(T)")) -> ()
        n243 = call <vilib>:"Add State(s) to Queue__jki_lib_state_machine.vi"("State(s) in Front (\"\")"=w469, "State(s) in (\"\")"=w478) -> ("States Out"=w477:string)  [unwired: 13 in]
      }
    }
  }
  n244 = call-dynamic "Cleanup.vi"("MenuStrip in"=w7) -> ()  [unwired: 10 in, 1 out]
